vi "SaccadeAnalyser - Main.vi"(8 "error in (no error)":errorcluster, 11 "Data IN":T3={"Impulse Positions"=[{"Start"=5471, "End"=5813, "Impulse Plane"=enum."Yaw", "Impulse Direction +ve?"=FALSE, "Time offset"=0, "Amplitude offset"=0.0}, {"Start"=6974, "End"=7325, "Impulse Plane"=enum."Yaw", "Impulse Direction +ve?"=TRUE, "Time offset"=0, "Amplitude offset"=0.0}, {"Start"=7641, "End"=7980, "Impulse Plane"=enum."Yaw", "Impulse Direction +ve?"=FALSE, "Time offset"=0, "Amplitude offset"=0.0}, {"Start"=9060, "End"=9400, "Impulse Plane"=enum."Yaw", "Impulse Direction +ve?"=FALSE, "Time offset"=0, "Amplitude offset"=0.0}, {"Start"=9938, "End"=10282, "Impulse Plane"=enum."Yaw", "Impulse Direction +ve?"=FALSE, "Time offset"=0, "Amplitude offset"=0.0}, {"Start"=10800, "End"=11142, "Impulse Plane"=enum."Yaw", "Impulse Direction +ve?"=FALSE, "Time offset"=0, "Amplitude offset"=0.0}, {"Start"=11602, "End"=11942, "Impulse Plane"=enum."Yaw", "Impulse Direction +ve?"=TRUE, "Time offset"=0, "Amplitude offset"=0.0}, {"Start"=12449, "End"=12790, "Impulse Plane"=enum."Yaw", "Impulse Direction +ve?"=TRUE, "Time offset"=0, "Amplitude offset"=0.0}, {"Start"=13310, "End"=13653, "Impulse Plane"=enum."Yaw", "Impulse Direction +ve?"=TRUE, "Time offset"=0, "Amplitude offset"=0.0}, {"Start"=14191, "End"=14535, "Impulse Plane"=enum."Yaw", "Impulse Direction +ve?"=TRUE, "Time offset"=0, "Amplitude offset"=0.0}, {"Start"=15040, "End"=15380, "Impulse Plane"=enum."Yaw", "Impulse Direction +ve?"=FALSE, "Time offset"=0, "Amplitude offset"=0.0}, {"Start"=16780, "End"=17124, "Impulse Plane"=enum."Yaw", "Impulse Direction +ve?"=TRUE, "Time offset"=0, "Amplitude offset"=0.0}, {"Start"=17572, "End"=17913, "Impulse Plane"=enum."Yaw", "Impulse Direction +ve?"=FALSE, "Time offset"=0, "Amplitude offset"=0.0}, {"Start"=18369, "End"=18713, "Impulse Plane"=enum."Yaw", "Impulse Direction +ve?"=FALSE, "Time offset"=0, "Amplitude offset"=0.0}, {"Start"=19174, "End"=19519, "Impulse Plane"=enum."Yaw", "Impulse Direction +ve?"=FALSE, "Time offset"=0, "Amplitude offset"=0.0}, {"Start"=19928, "End"=20270, "Impulse Plane"=enum."Yaw", "Impulse Direction +ve?"=TRUE, "Time offset"=0, "Amplitude offset"=0.0}, {"Start"=20762, "End"=21121, "Impulse Plane"=enum."Yaw", "Impulse Direction +ve?"=FALSE, "Time offset"=0, "Amplitude offset"=0.0}, {"Start"=21554, "End"=21888, "Impulse Plane"=enum."Yaw", "Impulse Direction +ve?"=FALSE, "Time offset"=0, "Amplitude offset"=0.0}, {"Start"=22293, "End"=22639, "Impulse Plane"=enum."Yaw", "Impulse Direction +ve?"=TRUE, "Time offset"=0, "Amplitude offset"=0.0}, {"Start"=23109, "End"=23464, "Impulse Plane"=enum."Yaw", "Impulse Direction +ve?"=TRUE, "Time offset"=0, "Amplitude offset"=0.0}, {"Start"=23868, "End"=24215, "Impulse Plane"=enum."Yaw", "Impulse Direction +ve?"=TRUE, "Time offset"=0, "Amplitude offset"=0.0}, {"Start"=24643, "End"=24992, "Impulse Plane"=enum."Yaw", "Impulse Direction +ve?"=FALSE, "Time offset"=0, "Amplitude offset"=0.0}, {"Start"=25685, "End"=26023, "Impulse Plane"=enum."Yaw", "Impulse Direction +ve?"=FALSE, "Time offset"=0, "Amplitude offset"=0.0}, {"Start"=26431, "End"=26768, "Impulse Plane"=enum."Yaw", "Impulse Direction +ve?"=FALSE, "Time offset"=0, "Amplitude offset"=0.0}, {"Start"=27251, "End"=27595, "Impulse Plane"=enum."Yaw", "Impulse Direction +ve?"=FALSE, "Time offset"=0, "Amplitude offset"=0.0}, {"Start"=28832, "End"=29180, "Impulse Plane"=enum."Yaw", "Impulse Direction +ve?"=TRUE, "Time offset"=0, "Amplitude offset"=0.0}, {"Start"=31028, "End"=31383, "Impulse Plane"=enum."LARP", "Impulse Direction +ve?"=FALSE, "Time offset"=0, "Amplitude offset"=0.0}, {"Start"=32603, "End"=32936, "Impulse Plane"=enum."LARP", "Impulse Direction +ve?"=TRUE, "Time offset"=0, "Amplitude offset"=0.0}, {"Start"=33445, "End"=33779, "Impulse Plane"=enum."LARP", "Impulse Direction +ve?"=TRUE, "Time offset"=0, "Amplitude offset"=0.0}, {"Start"=34276, "End"=34629, "Impulse Plane"=enum."LARP", "Impulse Direction +ve?"=FALSE, "Time offset"=0, "Amplitude offset"=0.0}, {"Start"=35114, "End"=35460, "Impulse Plane"=enum."LARP", "Impulse Direction +ve?"=FALSE, "Time offset"=0, "Amplitude offset"=0.0}, {"Start"=35981, "End"=36324, "Impulse Plane"=enum."LARP", "Impulse Direction +ve?"=TRUE, "Time offset"=0, "Amplitude offset"=0.0}, {"Start"=36920, "End"=37249, "Impulse Plane"=enum."LARP", "Impulse Direction +ve?"=TRUE, "Time offset"=0, "Amplitude offset"=0.0}, {"Start"=37988, "End"=38322, "Impulse Plane"=enum."LARP", "Impulse Direction +ve?"=TRUE, "Time offset"=0, "Amplitude offset"=0.0}, {"Start"=38964, "End"=39324, "Impulse Plane"=enum."LARP", "Impulse Direction +ve?"=FALSE, "Time offset"=0, "Amplitude offset"=0.0}, {"Start"=39948, "End"=40284, "Impulse Plane"=enum."LARP", "Impulse Direction +ve?"=TRUE, "Time offset"=0, "Amplitude offset"=0.0}, {"Start"=40958, "End"=41293, "Impulse Plane"=enum."LARP", "Impulse Direction +ve?"=TRUE, "Time offset"=0, "Amplitude offset"=0.0}, {"Start"=41899, "End"=42229, "Impulse Plane"=enum."LARP", "Impulse Direction +ve?"=TRUE, "Time offset"=0, "Amplitude offset"=0.0}, {"Start"=42801, "End"=43154, "Impulse Plane"=enum."LARP", "Impulse Direction +ve?"=FALSE, "Time offset"=0, "Amplitude offset"=0.0}, {"Start"=43641, "End"=43980, "Impulse Plane"=enum."LARP", "Impulse Direction +ve?"=TRUE, "Time offset"=0, "Amplitude offset"=0.0}, {"Start"=44466, "End"=44821, "Impulse Plane"=enum."LARP", "Impulse Direction +ve?"=FALSE, "Time offset"=0, "Amplitude offset"=0.0}, {"Start"=45388, "End"=45722, "Impulse Plane"=enum."LARP", "Impulse Direction +ve?"=TRUE, "Time offset"=0, "Amplitude offset"=0.0}, {"Start"=46149, "End"=46510, "Impulse Plane"=enum."LARP", "Impulse Direction +ve?"=FALSE, "Time offset"=0, "Amplitude offset"=0.0}, {"Start"=47874, "End"=48206, "Impulse Plane"=enum."LARP", "Impulse Direction +ve?"=TRUE, "Time offset"=0, "Amplitude offset"=0.0}, {"Start"=50143, "End"=50479, "Impulse Plane"=enum."RALP", "Impulse Direction +ve?"=TRUE, "Time offset"=0, "Amplitude offset"=0.0}, {"Start"=50976, "End"=51310, "Impulse Plane"=enum."RALP", "Impulse Direction +ve?"=FALSE, "Time offset"=0, "Amplitude offset"=0.0}, {"Start"=51892, "End"=52226, "Impulse Plane"=enum."RALP", "Impulse Direction +ve?"=FALSE, "Time offset"=0, "Amplitude offset"=0.0}, {"Start"=52839, "End"=53171, "Impulse Plane"=enum."RALP", "Impulse Direction +ve?"=FALSE, "Time offset"=0, "Amplitude offset"=0.0}, {"Start"=53676, "End"=54012, "Impulse Plane"=enum."RALP", "Impulse Direction +ve?"=TRUE, "Time offset"=0, "Amplitude offset"=0.0}, {"Start"=54530, "End"=54877, "Impulse Plane"=enum."RALP", "Impulse Direction +ve?"=FALSE, "Time offset"=0, "Amplitude offset"=0.0}, {"Start"=55371, "End"=55711, "Impulse Plane"=enum."RALP", "Impulse Direction +ve?"=TRUE, "Time offset"=0, "Amplitude offset"=0.0}, {"Start"=56153, "End"=56482, "Impulse Plane"=enum."RALP", "Impulse Direction +ve?"=FALSE, "Time offset"=0, "Amplitude offset"=0.0}, {"Start"=57053, "End"=57390, "Impulse Plane"=enum."RALP", "Impulse Direction +ve?"=FALSE, "Time offset"=0, "Amplitude offset"=0.0}, {"Start"=57954, "End"=58292, "Impulse Plane"=enum."RALP", "Impulse Direction +ve?"=FALSE, "Time offset"=0, "Amplitude offset"=0.0}, {"Start"=58794, "End"=59130, "Impulse Plane"=enum."RALP", "Impulse Direction +ve?"=TRUE, "Time offset"=0, "Amplitude offset"=0.0}, {"Start"=59587, "End"=59931, "Impulse Plane"=enum."RALP", "Impulse Direction +ve?"=TRUE, "Time offset"=0, "Amplitude offset"=0.0}, {"Start"=60399, "End"=60744, "Impulse Plane"=enum."RALP", "Impulse Direction +ve?"=FALSE, "Time offset"=0, "Amplitude offset"=0.0}, {"Start"=61218, "End"=61559, "Impulse Plane"=enum."RALP", "Impulse Direction +ve?"=FALSE, "Time offset"=0, "Amplitude offset"=0.0}, {"Start"=62100, "End"=62442, "Impulse Plane"=enum."RALP", "Impulse Direction +ve?"=FALSE, "Time offset"=0, "Amplitude offset"=0.0}, {"Start"=62989, "End"=63322, "Impulse Plane"=enum."RALP", "Impulse Direction +ve?"=FALSE, "Time offset"=0, "Amplitude offset"=0.0}, {"Start"=63787, "End"=64136, "Impulse Plane"=enum."RALP", "Impulse Direction +ve?"=TRUE, "Time offset"=0, "Amplitude offset"=0.0}, {"Start"=64603, "End"=64953, "Impulse Plane"=enum."RALP", "Impulse Direction +ve?"=FALSE, "Time offset"=0, "Amplitude offset"=0.0}, {"Start"=65462, "End"=65795, "Impulse Plane"=enum."RALP", "Impulse Direction +ve?"=FALSE, "Time offset"=0, "Amplitude offset"=0.0}, {"Start"=66308, "End"=66645, "Impulse Plane"=enum."RALP", "Impulse Direction +ve?"=FALSE, "Time offset"=0, "Amplitude offset"=0.0}, {"Start"=67052, "End"=67402, "Impulse Plane"=enum."RALP", "Impulse Direction +ve?"=TRUE, "Time offset"=0, "Amplitude offset"=0.0}], "No. Imp"=15, "Parameter Time Series"=[{"time offset"=0.0, "Offset"=0.0, "Gain"=1.0, "inverse"=FALSE, "filter data"=FALSE, "dots"=FALSE, "interpolate"=FALSE, "List 1"=5, "Color Box"=6618880, "Boolean"=TRUE}, {"time offset"=0.0, "Offset"=0.0, "Gain"=1.0, "inverse"=FALSE, "filter data"=FALSE, "dots"=FALSE, "interpolate"=FALSE, "List 1"=6, "Color Box"=6618880, "Boolean"=FALSE}, {"time offset"=0.0, "Offset"=0.0, "Gain"=1.0, "inverse"=FALSE, "filter data"=FALSE, "dots"=FALSE, "interpolate"=FALSE, "List 1"=7, "Color Box"=6618880, "Boolean"=FALSE}, {"time offset"=0.0, "Offset"=0.0, "Gain"=1.0, "inverse"=FALSE, "filter data"=FALSE, "dots"=FALSE, "interpolate"=FALSE, "List 1"=13, "Color Box"=16777224, "Boolean"=TRUE}, {"time offset"=0.0, "Offset"=0.0, "Gain"=1.0, "inverse"=FALSE, "filter data"=FALSE, "dots"=FALSE, "interpolate"=FALSE, "List 1"=14, "Color Box"=16777224, "Boolean"=FALSE}, {"time offset"=0.0, "Offset"=0.0, "Gain"=1.0, "inverse"=FALSE, "filter data"=FALSE, "dots"=FALSE, "interpolate"=FALSE, "List 1"=15, "Color Box"=16777224, "Boolean"=FALSE}], "Parameter Impuls Series"=[{"Color"=6618880, "Visible"=TRUE, "Channel"=1, "Invert"=FALSE, "Desaccade"=FALSE, "Offset"=0.0, "Gain"=1.0}, {"Color"=6618880, "Visible"=FALSE, "Channel"=6, "Invert"=FALSE, "Desaccade"=FALSE, "Offset"=0.0, "Gain"=1.0}, {"Color"=6618880, "Visible"=FALSE, "Channel"=7, "Invert"=FALSE, "Desaccade"=FALSE, "Offset"=0.0, "Gain"=1.0}, {"Color"=16777224, "Visible"=TRUE, "Channel"=13, "Invert"=FALSE, "Desaccade"=FALSE, "Offset"=0.0, "Gain"=1.0}, {"Color"=16777224, "Visible"=FALSE, "Channel"=14, "Invert"=FALSE, "Desaccade"=FALSE, "Offset"=0.0, "Gain"=1.0}, {"Color"=16777224, "Visible"=FALSE, "Channel"=15, "Invert"=FALSE, "Desaccade"=FALSE, "Offset"=0.0, "Gain"=1.0}], "Experiment Parameters"={"Freq"=0.0, "Vel"=0, "Acc"=0, "Stimulus"="Head Impulse"}, "Autosort File"=refnum, "Data File"={"Data Channels"=array34x71049[2415666 elements], "Sample Rate"=500, "Channel List"=["Hz Position-in-Head", "Hz Velocity-in-Head", "Hy Position-in-Head", "Hy Velocity-in-Head", "Hx Position-in-Head", "Hx Velocity-in-Head", "Hl Velocity-in-Head", "Hr Velocity-in-Head", "Lx Position-in-Head", "Ly Position-in-Head", "Lz Position-in-Head", "Lx Velocity-in-Head", "Ly Velocity-in-Head", "Lz Velocity-in-Head", "Ll Velocity-in-Head", "Lr Velocity-in-Head", "Rx Position-in-Head", "Ry Position-in-Head", "Rz Position-in-Head", "Rx Velocity-in-Head", "Ry Velocity-in-Head", "Rz Velocity-in-Head", "Rl Velocity-in-Head", "Rr Velocity-in-Head", "Target on/off", "aux input 1", "aux input 2", " ", "", "", "", "Target Hor", "Target Ver", ""]}, "Experiment data path"=path "C:/Users/w.figtree/Desktop/Coils Data/3", "Image data path"=path "/Macintosh HD/Users/patrick/Studium/Diploma Thesis/Data Analysis", "LVS data path"=path "/Macintosh HD/Users/patrick/Studium/Diploma Thesis/Data Analysis", "Raw copy path"=path "/Macintosh HD/Users/patrick/Studium/Diploma Thesis/Data Analysis", "filename"="passive_lvs.lvs", "desaccading parameters"={"Tolerance"=3, "Acc Range"=7000.0, "Sample Rate"=500, "Impulse Plane 2"=enum."Yaw", "Impulse dir"=FALSE}, "Experiment Parameters 2"={"Subject"="SE Trial Short Term", "Strain"="", "Rotation plane"="", "Experimenter"=" ", "Trial"=0.0, "Time"=0.0}, "Excel"={"Excel._Application"=refnum, "Use Excel"=TRUE, "Worksheet SINE"=refnum, "Row SINE"=0, "Worksheet TRANS"=refnum, "Row TRANS"=0}, "Session Config File"=refnum, "Autosort Parameter Set"=4, "EMA Version"="EMA 2016a", "desacc "={"Threshold 1 [Acc]"=7000.0, "Threshold 2 [% of TH1]"=60, "tolerance"=3, "Search WD "=0.1, " always use TH2"=FALSE, "Range"=3.0, "Max time"=120.0, "Min time"=20.0, "Velocity Threshold"=150}, "Cycle Nr for Saccades"={"POS"=0, "NEG"=0}, "calibration name"="u_calibration_1_p00001s001_calib.mat", "Excel"=refnum} {"Parameter Time Series"."time offset" format="%.3f"; "Parameter Time Series"."Gain" format="%.1f"; "Parameter Time Series"."Offset" format="%.1f"; "Parameter Time Series"."List 1" items=["Motor-Pos", "Motor-Vel", "Lx Position-in-Head", "Ly Position-in-Head", "Lz Position-in-Head", "Lx Velocity-in-Head", "Ly Velocity-in-Head", "Lz Velocity-in-Head", "Ll Velocity-in-Head", "Lr Velocity-in-Head", "Lx Accel-in-Head", "Ly Accel-in-Head", "Lz Accel-in-Head", "Rx Position-in-Head", "Ry Position-in-Head", "Rz Position-in-Head", "Rx Velocity-in-Head", "Ry Velocity-in-Head", "Rz Velocity-in-Head", "Rl Velocity-in-Head", "Rr Velocity-in-Head", "Rx Accel-in-Head", "Ry Accel-in-Head", "Rz Accel-in-Head", "Global Trigger", "", "", ""]; "Parameter Impuls Series"."Gain" format="%.1f"; "Parameter Impuls Series"."Offset" format="%.1f"}) -> (0 "error out":errorcluster, 3 "Data OUT":T3={"Impulse Positions"=[{"Start"=5471, "End"=5813, "Impulse Plane"=enum."Yaw", "Impulse Direction +ve?"=FALSE, "Time offset"=0, "Amplitude offset"=0.0}, {"Start"=6974, "End"=7325, "Impulse Plane"=enum."Yaw", "Impulse Direction +ve?"=TRUE, "Time offset"=0, "Amplitude offset"=0.0}, {"Start"=7641, "End"=7980, "Impulse Plane"=enum."Yaw", "Impulse Direction +ve?"=FALSE, "Time offset"=0, "Amplitude offset"=0.0}, {"Start"=9060, "End"=9400, "Impulse Plane"=enum."Yaw", "Impulse Direction +ve?"=FALSE, "Time offset"=0, "Amplitude offset"=0.0}, {"Start"=9938, "End"=10282, "Impulse Plane"=enum."Yaw", "Impulse Direction +ve?"=FALSE, "Time offset"=0, "Amplitude offset"=0.0}, {"Start"=10800, "End"=11142, "Impulse Plane"=enum."Yaw", "Impulse Direction +ve?"=FALSE, "Time offset"=0, "Amplitude offset"=0.0}, {"Start"=11602, "End"=11942, "Impulse Plane"=enum."Yaw", "Impulse Direction +ve?"=TRUE, "Time offset"=0, "Amplitude offset"=0.0}, {"Start"=12449, "End"=12790, "Impulse Plane"=enum."Yaw", "Impulse Direction +ve?"=TRUE, "Time offset"=0, "Amplitude offset"=0.0}, {"Start"=13310, "End"=13653, "Impulse Plane"=enum."Yaw", "Impulse Direction +ve?"=TRUE, "Time offset"=0, "Amplitude offset"=0.0}, {"Start"=14191, "End"=14535, "Impulse Plane"=enum."Yaw", "Impulse Direction +ve?"=TRUE, "Time offset"=0, "Amplitude offset"=0.0}, {"Start"=15040, "End"=15380, "Impulse Plane"=enum."Yaw", "Impulse Direction +ve?"=FALSE, "Time offset"=0, "Amplitude offset"=0.0}, {"Start"=16780, "End"=17124, "Impulse Plane"=enum."Yaw", "Impulse Direction +ve?"=TRUE, "Time offset"=0, "Amplitude offset"=0.0}, {"Start"=17572, "End"=17913, "Impulse Plane"=enum."Yaw", "Impulse Direction +ve?"=FALSE, "Time offset"=0, "Amplitude offset"=0.0}, {"Start"=18369, "End"=18713, "Impulse Plane"=enum."Yaw", "Impulse Direction +ve?"=FALSE, "Time offset"=0, "Amplitude offset"=0.0}, {"Start"=19174, "End"=19519, "Impulse Plane"=enum."Yaw", "Impulse Direction +ve?"=FALSE, "Time offset"=0, "Amplitude offset"=0.0}, {"Start"=19928, "End"=20270, "Impulse Plane"=enum."Yaw", "Impulse Direction +ve?"=TRUE, "Time offset"=0, "Amplitude offset"=0.0}, {"Start"=20762, "End"=21121, "Impulse Plane"=enum."Yaw", "Impulse Direction +ve?"=FALSE, "Time offset"=0, "Amplitude offset"=0.0}, {"Start"=21554, "End"=21888, "Impulse Plane"=enum."Yaw", "Impulse Direction +ve?"=FALSE, "Time offset"=0, "Amplitude offset"=0.0}, {"Start"=22293, "End"=22639, "Impulse Plane"=enum."Yaw", "Impulse Direction +ve?"=TRUE, "Time offset"=0, "Amplitude offset"=0.0}, {"Start"=23109, "End"=23464, "Impulse Plane"=enum."Yaw", "Impulse Direction +ve?"=TRUE, "Time offset"=0, "Amplitude offset"=0.0}, {"Start"=23868, "End"=24215, "Impulse Plane"=enum."Yaw", "Impulse Direction +ve?"=TRUE, "Time offset"=0, "Amplitude offset"=0.0}, {"Start"=24643, "End"=24992, "Impulse Plane"=enum."Yaw", "Impulse Direction +ve?"=FALSE, "Time offset"=0, "Amplitude offset"=0.0}, {"Start"=25685, "End"=26023, "Impulse Plane"=enum."Yaw", "Impulse Direction +ve?"=FALSE, "Time offset"=0, "Amplitude offset"=0.0}, {"Start"=26431, "End"=26768, "Impulse Plane"=enum."Yaw", "Impulse Direction +ve?"=FALSE, "Time offset"=0, "Amplitude offset"=0.0}, {"Start"=27251, "End"=27595, "Impulse Plane"=enum."Yaw", "Impulse Direction +ve?"=FALSE, "Time offset"=0, "Amplitude offset"=0.0}, {"Start"=28832, "End"=29180, "Impulse Plane"=enum."Yaw", "Impulse Direction +ve?"=TRUE, "Time offset"=0, "Amplitude offset"=0.0}, {"Start"=31028, "End"=31383, "Impulse Plane"=enum."LARP", "Impulse Direction +ve?"=FALSE, "Time offset"=0, "Amplitude offset"=0.0}, {"Start"=32603, "End"=32936, "Impulse Plane"=enum."LARP", "Impulse Direction +ve?"=TRUE, "Time offset"=0, "Amplitude offset"=0.0}, {"Start"=33445, "End"=33779, "Impulse Plane"=enum."LARP", "Impulse Direction +ve?"=TRUE, "Time offset"=0, "Amplitude offset"=0.0}, {"Start"=34276, "End"=34629, "Impulse Plane"=enum."LARP", "Impulse Direction +ve?"=FALSE, "Time offset"=0, "Amplitude offset"=0.0}, {"Start"=35114, "End"=35460, "Impulse Plane"=enum."LARP", "Impulse Direction +ve?"=FALSE, "Time offset"=0, "Amplitude offset"=0.0}, {"Start"=35981, "End"=36324, "Impulse Plane"=enum."LARP", "Impulse Direction +ve?"=TRUE, "Time offset"=0, "Amplitude offset"=0.0}, {"Start"=36920, "End"=37249, "Impulse Plane"=enum."LARP", "Impulse Direction +ve?"=TRUE, "Time offset"=0, "Amplitude offset"=0.0}, {"Start"=37988, "End"=38322, "Impulse Plane"=enum."LARP", "Impulse Direction +ve?"=TRUE, "Time offset"=0, "Amplitude offset"=0.0}, {"Start"=38964, "End"=39324, "Impulse Plane"=enum."LARP", "Impulse Direction +ve?"=FALSE, "Time offset"=0, "Amplitude offset"=0.0}, {"Start"=39948, "End"=40284, "Impulse Plane"=enum."LARP", "Impulse Direction +ve?"=TRUE, "Time offset"=0, "Amplitude offset"=0.0}, {"Start"=40958, "End"=41293, "Impulse Plane"=enum."LARP", "Impulse Direction +ve?"=TRUE, "Time offset"=0, "Amplitude offset"=0.0}, {"Start"=41899, "End"=42229, "Impulse Plane"=enum."LARP", "Impulse Direction +ve?"=TRUE, "Time offset"=0, "Amplitude offset"=0.0}, {"Start"=42801, "End"=43154, "Impulse Plane"=enum."LARP", "Impulse Direction +ve?"=FALSE, "Time offset"=0, "Amplitude offset"=0.0}, {"Start"=43641, "End"=43980, "Impulse Plane"=enum."LARP", "Impulse Direction +ve?"=TRUE, "Time offset"=0, "Amplitude offset"=0.0}, {"Start"=44466, "End"=44821, "Impulse Plane"=enum."LARP", "Impulse Direction +ve?"=FALSE, "Time offset"=0, "Amplitude offset"=0.0}, {"Start"=45388, "End"=45722, "Impulse Plane"=enum."LARP", "Impulse Direction +ve?"=TRUE, "Time offset"=0, "Amplitude offset"=0.0}, {"Start"=46149, "End"=46510, "Impulse Plane"=enum."LARP", "Impulse Direction +ve?"=FALSE, "Time offset"=0, "Amplitude offset"=0.0}, {"Start"=47874, "End"=48206, "Impulse Plane"=enum."LARP", "Impulse Direction +ve?"=TRUE, "Time offset"=0, "Amplitude offset"=0.0}, {"Start"=50143, "End"=50479, "Impulse Plane"=enum."RALP", "Impulse Direction +ve?"=TRUE, "Time offset"=0, "Amplitude offset"=0.0}, {"Start"=50976, "End"=51310, "Impulse Plane"=enum."RALP", "Impulse Direction +ve?"=FALSE, "Time offset"=0, "Amplitude offset"=0.0}, {"Start"=51892, "End"=52226, "Impulse Plane"=enum."RALP", "Impulse Direction +ve?"=FALSE, "Time offset"=0, "Amplitude offset"=0.0}, {"Start"=52839, "End"=53171, "Impulse Plane"=enum."RALP", "Impulse Direction +ve?"=FALSE, "Time offset"=0, "Amplitude offset"=0.0}, {"Start"=53676, "End"=54012, "Impulse Plane"=enum."RALP", "Impulse Direction +ve?"=TRUE, "Time offset"=0, "Amplitude offset"=0.0}, {"Start"=54530, "End"=54877, "Impulse Plane"=enum."RALP", "Impulse Direction +ve?"=FALSE, "Time offset"=0, "Amplitude offset"=0.0}, {"Start"=55371, "End"=55711, "Impulse Plane"=enum."RALP", "Impulse Direction +ve?"=TRUE, "Time offset"=0, "Amplitude offset"=0.0}, {"Start" (continued)
    shift-left: T6 {"Impulse Data"=refnum, "Sample Rate (Hz)"=0.0, "Num Impulses"=0, "Impulse Duration (samples)"=0, "Palette"={"Stimulus"=6618880, "Response"=16777224, "Saccade"=16777224, "Excluded Saccade"=16777224, "Sibling Saccade"=16777224, "Selected Saccade"=16777224}, "Saccades"=[], "Summary"={"Num Impulses"=0.0, "Num Saccades"=0.0, "Onset (ms)"=0.0, "Onset SD (ms)"=0.0, "Duration (ms)"=0.0, "Duration SD (ms)"=0.0, "Vel (°/s)"=0.0, "Vel SD (°/s)"=0.0, "Amplitude (°)"=0.0, "Amplitude SD (°)"=0.0, "Gain"=0.0, "Gain SD"=0.0}, "Group Summary"=[]} ("Saccade Analyser Data") -> [w121]
    stop <- w126 stop-if-true
    # "Main Loop"
    n86 = Dequeue Element(queue=w129) -> (queue out=w128:refnum<queue>, element=w127:T10)  [unwired: 2 in, 2 out]
    n87 = case shown="\"Export - Saccades\"" w127 {
      tunnel: w128 -> [_ w158 _ w180 w187 _ _ _ _ _ _ w464 _ _ _ _ _ _ _ _ _ _ _ _ _ w702 w709 w715 _ _ _ _ _ _ w900]
      tunnel: [_ _ TRUE _ _ _ _ _ _ _ _ _ _ _ _ _ _ _ _ _ _ _ _ _ _ _ _ _ _ _ _ _ _ _ _] -> w126
      tunnel: w125 -> [w132 w156 w177 w183 w190 w219 w236 w279 w328 w369 w409 w467 w473 w487 w521 w572 w598 w622 w661 w667 w673 w678 w685 w689 w696 w705 w712 w719 w724 w745 w773 w789 w829 w839 w904]
      tunnel: w124 -> [w131 w162 w176 w182 w189 w220 w235 w278 w327 w368 w408 w466 w472 w486 w520 w571 w597 w621 w660 w666 w672 w677 w684 w688 w695 w704 w711 w718 w733 w770 w782 w810 w837 w864 w903]
      tunnel: [w132 w156 w177 w183 w190 w219 w236 w279 w328 w369 w409 w467 w473 w487 w521 w572 w598 w622 w661 w667 w673 w678 w685 w689 w696 w705 w712 w719 w723 w744 w772 w790 w830 w841 w904] -> w123
      tunnel: [w131 w162 w176 w182 w189 w220 w235 w278 w327 w368 w408 w466 w472 w486 w520 w571 w597 w621 w660 w666 w672 w677 w684 w688 w695 w704 w711 w718 w733 w770 w782 w810 w837 w864 w903] -> w122
      tunnel: w121 -> [w130 w161 w175 w181 w188 w215 w234 w276 w326 w367 w405 w465 w471 w481 w508 w570 w596 w620 w658 w665 w671 w676 w683 w687 w692 w703 w710 w717 w722 w735 w771 w791 w828 w840 w902]
      tunnel: [w130 w160 w175 w181 w188 w213 w234 w275 w325 w366 w404 w465 w471 w481 w508 w570 w596 w620 w658 w665 w671 w676 w683 w687 w691 w703 w710 w717 w722 w735 w771 w791 w828 w840 w902] -> w120
      frame Default {
        # "Unhandled state. Should never occur."
        n88 = One Button Dialog(message="Error: Unhandled state in Saccade Analyser!") -> ()  [unwired: 1 in, 1 out]
      }
      frame "Initialise" {
        w137 = u16 10 items=["Hz Position-in-Head", "Hz Velocity-in-Head", "Hy Position-in-Head", "Hy Velocity-in-Head", "Hx Position-in-Head", "Hx Velocity-in-Head", "Hl Velocity-in-Head", "Hr Velocity-in-Head", "Lx Position-in-Head", "Ly Position-in-Head", "Lz Position-in-Head", "Lx Velocity-in-Head", "Ly Velocity-in-Head", "Lz Velocity-in-Head", "Ll Velocity-in-Head", "Lr Velocity-in-Head", "Rx Position-in-Head", "Ry Position-in-Head", "Rz Position-in-Head", "Rx Velocity-in-Head", "Ry Velocity-in-Head", "Rz Velocity-in-Head", "Rl Velocity-in-Head", "Rr Velocity-in-Head", "Target on/off", "aux input 1", "aux input 2", " ", "", "", "", "Target Hor", "Target Ver", ""] ("ring_response channel")
        w146 = u16 13 items=["Hz Position-in-Head", "Hz Velocity-in-Head", "Hy Position-in-Head", "Hy Velocity-in-Head", "Hx Position-in-Head", "Hx Velocity-in-Head", "Hl Velocity-in-Head", "Hr Velocity-in-Head", "Lx Position-in-Head", "Ly Position-in-Head", "Lz Position-in-Head", "Lx Velocity-in-Head", "Ly Velocity-in-Head", "Lz Velocity-in-Head", "Ll Velocity-in-Head", "Lr Velocity-in-Head", "Rx Position-in-Head", "Ry Position-in-Head", "Rz Position-in-Head", "Rx Velocity-in-Head", "Ry Velocity-in-Head", "Rz Velocity-in-Head", "Rl Velocity-in-Head", "Rr Velocity-in-Head", "Target on/off", "aux input 1", "aux input 2", " ", "", "", "", "Target Hor", "Target Ver", ""] ("ring_response channel")
        w145 = u16 1 items=["Hz Position-in-Head", "Hz Velocity-in-Head", "Hy Position-in-Head", "Hy Velocity-in-Head", "Hx Position-in-Head", "Hx Velocity-in-Head", "Hl Velocity-in-Head", "Hr Velocity-in-Head", "Lx Position-in-Head", "Ly Position-in-Head", "Lz Position-in-Head", "Lx Velocity-in-Head", "Ly Velocity-in-Head", "Lz Velocity-in-Head", "Ll Velocity-in-Head", "Lr Velocity-in-Head", "Rx Position-in-Head", "Ry Position-in-Head", "Rz Position-in-Head", "Rx Velocity-in-Head", "Ry Velocity-in-Head", "Rz Velocity-in-Head", "Rl Velocity-in-Head", "Rr Velocity-in-Head", "Target on/off", "aux input 1", "aux input 2", " ", "", "", "", "Target Hor", "Target Ver", ""] ("ring_stimulus channel")
        # "LARP and RALP position are unfortunately not included in EMAs default data set. Since this plugin needs this data it will calculate it from the xyz data. In order to present a unified interface the channels are included in the UI list here."
        # "Configure VI for execution."
        n89 = control-ref of="mclb_saccades"() -> (w138:refnum<vi>)
        n90 = Enqueue Element(queue=w158, element=Saccade_Analyser_States."DO - Analysis") -> ()  [unwired: 2 in, 3 out]
        n91 = local write "Tab Control"(enum32{"Channel Select", "Detection", "Gain"}."Channel Select" ("Tab Control")) -> ()
        n92 = local write "enum_direction"(enum16{"Positive", "Negative"}."Positive" ("enum_direction")) -> ()
        n93 = local write "enum_plane"(T14."Yaw" ("enum_plane")) -> ()
        n94 = property on="Property Node" class="MCListbox (strict)"(reference=w138, "Key Focus"=TRUE) -> ()  [unwired: 1 in, 2 out]
        n95 = local write "ring_stimulusChannel"(w145) -> ()
        n96 = local write "ring_responseChannel"(w146) -> ()
        n97 = local write "ring_responsePosChannel"(w137) -> ()
        n98 = disable-structure shown="Disabled" {
          frame Disabled {
            # "Initialise analysis configuration. Disabled to allow value persistence between dialog calls."
            n99 = local write "sac_NSampleTime"(u32 10 ("sac_NSamples")) -> ()
            n100 = local write "bool_includePrePeak"(TRUE ("bool_includePrePeak")) -> ()
            n101 = local write "stim_Onset%"(4.0 ("Impulse Onset %")) -> ()
            n102 = local write "sac_BiphasicCond"(1.5 ("sac_BiphasicCond")) -> ()
            n103 = local write "sac_AccMult"(1.3 ("sac_AccMult")) -> ()
            n104 = local write "sac_AccMin"(2000.0 ("sac_AccMin")) -> ()
            n105 = local write "bool_autoChannel"(TRUE ("bool_autoChannel")) -> ()
            n106 = local write "enum_summaryType"(enum16{"Mean", "Median"}."Mean" ("enum_summaryType")) -> ()
            n107 = local write "gain_WinDur"(30.0 ("gain_WinDur")) -> ()
            n108 = local write "gain_WinLead"(40.0 ("gain_WinLead")) -> ()
            n109 = local write "gain_Valid%"(50.0 ("gain_ Valid%")) -> ()
          }
          frame Enabled {
          }
        }
        n110 = Unbundle By Name(w156) -> ("Data File.Sample Rate"=w159:i32, "Data File.Channel List"=w136:string[])
        n111 = Build Array (concatenate)(w136, string[] ["Ll Position-in-Head", "Lr Position-in-Head"] ("element")) -> (w135:string[])
        n112 = property on="ring_stimulusChannel" class="Ring (strict)"("Strings []"=w135) -> ()  [unwired: 2 in, 2 out]
        n113 = property on="ring_responsePosChannel" class="Ring (strict)"("Strings []"=w135) -> ()  [unwired: 2 in, 2 out]
        n114 = property on="ring_responseChannel" class="Ring (strict)"("Strings []"=w135) -> ()  [unwired: 2 in, 2 out]
        n115 = Bundle By Name(cluster=T7 {"Stimulus"=6618880, "Response"=16777224, "Saccade"=16777224, "Excluded Saccade"=16777224, "Sibling Saccade"=16777224, "Selected Saccade"=16777224} ("Palette"), "Stimulus"=u32 122893, "Response"=u32 16777224, "Saccade"=u32 16728128, "Excluded Saccade"=u32 9868950, "Sibling Saccade"=u32 16728128, "Selected Saccade"=u32 16728128) -> (w143:T7)
        n116 = New Data Value Reference(data value=T15[] []) -> (data value reference=w151:refnum<data-value>)  [unwired: 1 in, 1 out]
        n117 = Bundle By Name(cluster=w161, "Impulse Data"=w151, "Sample Rate (Hz)"=w159, "Palette"=w143, "Saccades"=T8[] []) -> (w160:T6)
      }
      frame "Quit" {
        # "End VI execution."
        n118 = Unbundle By Name(w175) -> ("Impulse Data"=w174:refnum<data-value>)
        n119 = Delete Data Value Reference(data value reference=w174) -> ()  [unwired: 1 in, 2 out]
      }
      frame "DO - Analysis" {
        w179 = T10[] [enum."Halt Panel Updates", enum."Disable Controls", enum."Load Channel Data", enum."Find Impulses", enum."Find Saccades", enum."Sequence Saccades", enum."Calc Saccade Summary Stats", enum."Calc Saccade Group Stats", enum."DO - Draw"] items=["Initialise", "Quit", "DO - Analysis", "DO - Summary Analysis", "Load Channel Data", "Find Impulses", "Find Saccades", "Sequence Saccades", "Calc Saccade Summary Stats", "Calc Saccade Group Stats", "DO - Draw", "Clear Plot", "Plot Selected Saccade", "Plot Selected Saccade Siblings", "Plot Impulse Data", "Plot Saccade Data", "Fill Saccade MCLB", "Fill Summary Stats", "Give MCLB Focus", "Halt Panel Updates", "Resume Panel Updates", "Disable Controls", "Enable Controls", "Toggle Saccade", "DO - Export Summary", "Export - Open Summary", "Export - Summary", "DO - Export Saccades", "Export - Open Saccades", "Export - Saccades", "DO - Export Group", "Export - Open Group", "Export - Group", "Do - Export All"] ("element")
        # "Enqueue analysis process states."
        n120 = for {
          tunnel: w180 -> [w185]
          tunnel: w179 -> [w184] mode=indexing
          n121 = Enqueue Element(queue=w185, element=w184) -> ()  [unwired: 2 in, 3 out]
        }
      }
      frame "DO - Summary Analysis" {
        w186 = T10[] [enum."Halt Panel Updates", enum."Disable Controls", enum."Sequence Saccades", enum."Calc Saccade Summary Stats", enum."Calc Saccade Group Stats", enum."DO - Draw"] items=["Initialise", "Quit", "DO - Analysis", "DO - Summary Analysis", "Load Channel Data", "Find Impulses", "Find Saccades", "Sequence Saccades", "Calc Saccade Summary Stats", "Calc Saccade Group Stats", "DO - Draw", "Clear Plot", "Plot Selected Saccade", "Plot Selected Saccade Siblings", "Plot Impulse Data", "Plot Saccade Data", "Fill Saccade MCLB", "Fill Summary Stats", "Give MCLB Focus", "Halt Panel Updates", "Resume Panel Updates", "Disable Controls", "Enable Controls", "Toggle Saccade", "DO - Export Summary", "Export - Open Summary", "Export - Summary", "DO - Export Saccades", "Export - Open Saccades", "Export - Saccades", "DO - Export Group", "Export - Open Group", "Export - Group", "Do - Export All"] ("element")
        # "Enqueue only the summary analysis process states."
        n122 = for {
          tunnel: w187 -> [w192]
          tunnel: w186 -> [w191] mode=indexing
          n123 = Enqueue Element(queue=w192, element=w191) -> ()  [unwired: 2 in, 3 out]
        }
      }
      frame "Load Channel Data" {
        # "Build Impulse Filter"
        # "Get Impulse Data"
        # "Load channel data from Data IN and sort them into impulses."
        n124 = property on="ring_responsePosChannel" class="Ring (strict)"() -> ("Strings []"=w195:string[], "Value"=w196:u16)  [unwired: 2 in, 2 out]
        n125 = property on="ring_stimulusChannel" class="Ring (strict)"() -> ("Strings []"=w207:string[], "Value"=w206:u16)  [unwired: 2 in, 2 out]
        n126 = property on="ring_responseChannel" class="Ring (strict)"() -> ("Strings []"=w205:string[], "Value"=w204:u16)  [unwired: 2 in, 2 out]
        n127 = local read "enum_direction"() -> (w211:enum16{"Positive", "Negative"})
        n128 = local read "enum_plane"() -> (w208:T2)
        n129 = Index Array(array=w207, index=w206) -> (element=w203:string)
        n130 = Index Array(array=w195, index=w196) -> (element=w194:string)
        n131 = Index Array(array=w205, index=w204) -> (element=w202:string)
        n132 = Build Array(w203, w202, w194) -> (w201:string[])
        n133 = Equal To 0?(x=w211) -> (x = 0?=w210:bool)
        n134 = Bundle By Name(cluster=T16 {"Channels"=["Hz Velocity-in-Head", "Lz Velocity-in-Head"], "Impulse Plane"=enum."Yaw", "Impulse Direction +ve?"=TRUE} ("Impulse Select"), "Channels"=w201, "Impulse Plane"=w208, "Impulse Direction +ve?"=w210) -> (w209:T16)
        n135 = Unbundle By Name(w219) -> ("Data File"=w218:T19, "Impulse Positions"=w217:T20)
        n136 = local read "bool_isCoilsData"() -> (w193:bool)
        n137 = call "Sort Impulses.vi"("Is Coils Data?"=w193, "Impulse Select"=w209, "Impulse Positions"=w217, "Data Input"=w218) -> ("Num Impulses"=w198:i32, "Impulses Duration (samples)"=w197:i32, "Impulse Data"=w200:dbl[][])  [unwired: 4 in, 1 out]
        n138 = for {
          N: w198 -> [_]
          tunnel: w200 -> [w229]
          tunnel: w198 -> [w221]
          tunnel: [w227] -> w199 mode=indexing
          i -> [w223]
          # "Collect data into impulse clusters\nData is organised by row first by impulse index then by channel index."
          n139 = Add(x=w223, y=w221) -> (x+y=w222:i32)
          n140 = Add(x=w222, y=w221) -> (x+y=w224:i32)
          n141 = Index Array(array=w229, index (row) #1=w223, index (row) #2=w222, index (row) #3=w224) -> (element #1=w228:dbl[], element #2=w226:dbl[], element #3=w225:dbl[])  [unwired: 3 in]
          n142 = Bundle By Name(cluster=T15 {"Stimulus Data"=[], "Response Data"=[], "Response Pos Data"=[], "Peak (idx)"=0, "Onset (idx)"=0} ("Impulse"), "Stimulus Data"=w228, "Response Data"=w226, "Response Pos Data"=w225) -> (w227:T15)
        }
        n143 = Unbundle By Name(w215) -> ("Impulse Data"=w216:refnum<data-value>)
        n144 = in-place {
          in-place-border: w199 -> [w231]
          n145 = in-place-dvr #1(w216) -> ()  [unwired: 2 out]
          n146 = in-place-dvr #1(w231) -> (w214:refnum<data-value>)  [unwired: 1 out]
        }
        n147 = Bundle By Name(cluster=w215, "Num Impulses"=w198, "Impulse Duration (samples)"=w197, "Impulse Data"=w214) -> (w213:T6)
      }
      frame "Find Impulses" {
        # "Finds the onset and peak of each impulse."
        n148 = Unbundle By Name(w234) -> ("Impulse Data"=w233:refnum<data-value>)
        n149 = local read "enum_direction"() -> (w232:enum16{"Positive", "Negative"})
        n150 = in-place {
          in-place-border: w232 -> [w237]
          n151 = in-place-dvr #2(w233) -> (w239:T15[])  [unwired: 1 out]
          n152 = for {
            tunnel: w239 -> [w246] mode=indexing
            tunnel: [w245] -> w238 mode=indexing
            tunnel: w237 -> [w241]
            # "Smooth signal"
            # "Find onset"
            # "Find Peak"
            # "For each impulse..."
            n153 = Unbundle By Name(w246) -> ("Stimulus Data"=w242:dbl[])
            n154 = call "SaccadeAnalyser - Make Traces Positive.vi"("enum_direction"=w241, "Stimulus in"=w242) -> ("Stimulus out"=w240:dbl[])  [unwired: 7 in, 2 out]
            n155 = Array Max & Min(array=w240) -> (max value=w253:dbl, max index (indices)=w244:i32)  [unwired: 2 out]
            n156 = local read "stim_Onset%"() -> (w255:dbl)
            n157 = call <vilib>:"Median Filter.vi"("left rank"=10, "X"=w240) -> ("Filtered X"=w248:dbl[])  [unwired: 8 in, 1 out]
            n158 = Divide(x=w255, y=100.0) -> (x/y=w252:dbl)
            n159 = Multiply(x=w253, y=w252) -> (x*y=w251:dbl)
            n160 = Greater?(x=w248, y=w251) -> (0:w250:bool[])
            n161 = Search 1D Array(1D array=w250, element=TRUE) -> (index of element=w243:i32)  [unwired: 1 in]
            n162 = Bundle By Name(cluster=w246, "Peak (idx)"=w244, "Onset (idx)"=w243) -> (w245:T15)
          }
          n163 = in-place-dvr #2(w238) -> ()  [unwired: 2 out]
        }
      }
      frame "Find Saccades" {
        # "Finds the saccades within each impulse and calculates the saccade onset, peak, duration, etc..."
        n164 = local read "enum_direction"() -> (w269:enum16{"Positive", "Negative"})
        n165 = Unbundle By Name(w276) -> ("Impulse Data"=w277:refnum<data-value>, "Sample Rate (Hz)"=w265:dbl)
        n166 = in-place {
          in-place-border: w265 -> [w283]
          in-place-border: [w282] -> w274
          in-place-border: w269 -> [w281]
          n167 = in-place-dvr #3(w277) -> (w285:T15[])  [unwired: 1 out]
          n168 = for {
            tunnel: w285 -> [w303] mode=indexing
            tunnel: [w303] -> w284 mode=indexing
            tunnel: w283 -> [w289]
            tunnel: [w301] -> w282 mode=concatenating
            tunnel: w281 -> [w300]
            i -> [w302]
            # "For each impulse..."
            n169 = Unbundle By Name(w303) -> ("Peak (idx)"=w286:i32, "Onset (idx)"=w298:i32, "Response Data"=w299:dbl[])
            n170 = local read "sac_NSampleTime"() -> (w294:dbl)
            n171 = local read "sac_BiphasicCond"() -> (w295:dbl)
            n172 = local read "bool_includePrePeak"() -> (w287:bool)
            n173 = local read "sac_AccMult"() -> (w296:dbl)
            n174 = local read "sac_AccMin"() -> (w297:dbl)
            n175 = Divide(x=w294, y=1000.0) -> (x/y=w293:dbl)
            n176 = call "SaccadeAnalyser - Make Traces Positive.vi"("enum_direction"=w300, "Response in"=w299) -> ("Response out"=w290:dbl[])  [unwired: 7 in, 2 out]
            n177 = Bundle(w293, "sac_AccMin"=w297, "sac_AccMult"=w296, "sac_BiphasicCond"=w295) -> (w288:T21)  [unwired: 1 in]
            n178 = call "Detect Saccades 2.vi"("Config"=w288, "Sample Rate (Hz)"=w289, "Velocity Data"=w290) -> ("Saccades"=w291:T8[])  [unwired: 7 in, 1 out]
            n179 = for {
              tunnel: [w315] -> w301 mode=indexing if=w309
              tunnel: w302 -> [w311]
              tunnel: w291 -> [w313] mode=indexing
              tunnel: w298 -> [w312]
              tunnel: w287 -> [w305]
              tunnel: w286 -> [w307]
              # "Check saccade is post onset"
              # "Check saccade is post peak"
              # "Remove early saccades and fill in basic info"
              n180 = Unbundle By Name(w313) -> ("Start (idx)"=w308:dbl)
              n181 = Bundle By Name(cluster=w313, "Impulse"=w311, "Included?"=TRUE) -> (w315:T8)
              n182 = Greater?(x=w308, y=w312) -> (0:w310:bool)
              n183 = Greater?(x=w308, y=w307) -> (0:w306:bool)
              n184 = Compound Arithmetic op=OR(w305, w306) -> (w304:bool)
              n185 = Compound Arithmetic op=AND(w304, w310) -> (w309:bool)
            }
          }
          n186 = in-place-dvr #3(w284) -> (w266:refnum<data-value>, w280:errorcluster)
        }
        n187 = call "Detect Saccade Peak.vi"("enum_direction"=w269, "Impulse Data"=w266, "error in (no error)"=w280, "Saccades in"=w274) -> ("error out"=w272:errorcluster, "Saccade out"=w273:T8[])  [unwired: 4 in]
        n188 = call "Trim Saccade Tail for Symmetry.vi"("error in (no error)"=w272, "Saccades in"=w273) -> ("error out"=w270:errorcluster, "Saccades out"=w271:T8[])  [unwired: 8 in]
        n189 = local read "gain_WinLead"() -> (w260:dbl)
        n190 = local read "gain_WinDur"() -> (w259:dbl)
        n191 = local read "gain_Valid%"() -> (w263:dbl)
        n192 = Bundle("gain_WinLead"=w260, "gain_WinDur"=w259) -> (w258:cluster{"gain_WinLead":dbl, "gain_WinDur":dbl})  [unwired: 1 in]
        n193 = call "Calculate Saccade Parameters.vi"("Impulse Data"=w266, "error in (no error)"=w270, "Sample Rate (Hz)"=w265, "enum_direction"=w269, "Saccades in"=w271) -> ("error out"=w267:errorcluster, "Saccade out"=w268:T8[])  [unwired: 5 in]
        n194 = Divide(x=w263, y=100.0) -> (x/y=w261:dbl)
        n195 = Divide(x=w258, y=1000.0) -> (x/y=w256:cluster{"gain_WinLead":dbl, "gain_WinDur":dbl})
        n196 = call "Calculate Saccade Gain.vi"("Gain Window"=w256, "Impulse Data"=w266, "error in (no error)"=w267, "Sample Rate (Hz)"=w265, "Valid Range Fraction"=w261, "Saccades in"=w268) -> ("Saccade out"=w264:T8[])  [unwired: 4 in, 1 out]
        n197 = Bundle By Name(cluster=w276, "Saccades"=w264) -> (w275:T6)
      }
      frame "Sequence Saccades" {
        w323 = u16 0 items=["Real, Imaginary", "Magnitude, Real, Imaginary", "Magnitude, Phase Angle"] ("method")
        # "Sort array. First by Impulse number (real) and then by onset index (imaginary)."
        # "Determines the order in which saccades appear within an impulse."
        n198 = Unbundle By Name(w326) -> ("Saccades"=w322:T8[])
        n199 = for {
          tunnel: w322 -> [w345] mode=indexing
          tunnel: [w343] -> w321 mode=indexing
          # "Initialise sequence number to NaN."
          n200 = Bundle By Name(cluster=w345, "Sequence #"=nan) -> (w343:T8)
        }
        n201 = for {
          tunnel: w321 -> [w351] mode=indexing
          tunnel: [w348] -> w324 mode=indexing if=w346
          tunnel: [w347] -> w320 mode=indexing if=w346
          i -> [w347]
          # "Get included saccades and build sorting array."
          n202 = Unbundle By Name(w351) -> ("Impulse"=w350:i32, "Start (idx)"=w349:dbl, "Included?"=w346:bool)
          n203 = Re/Im To Complex(1:w349, 2:w350) -> (0:w348:cdb)
        }
        n204 = call <vilib>:"Sort Complex Numbers.vi"("method"=w323, "Complex Numbers"=w324) -> ("Sorted Index"=w319:i32[])  [unwired: 7 in, 2 out]
        n205 = call-poly <userlib>:"Reorder Array2__ogtk.vi"("indices"=w319, "array"=w320) -> ("reordered array"=w318:i32[])  [unwired: 9 in]
        n206 = for {
          tunnel: w318 -> [w332] mode=indexing
          shift-right: [w331] -> w317
          shift-left: w321 -> [w333]
          shift-right: [FALSE] -> _
          shift-left: TRUE -> [w330]
          # "For each ordered and included saccade determine the sequence number"
          n207 = in-place {
            in-place-border: w330 -> [w334]
            n208 = in-place-array #4(w333, w332) -> (w340:T8)
            n209 = Unbundle By Name(w340) -> ("Impulse"=w342:i32)
            n210 = call-poly <userlib>:"Data Changed__ogtk.vi"("I32"=w342) -> ("Changed"=w336:bool)
            n211 = Compound Arithmetic op=OR(w336, w334) -> (w335:bool)
            n212 = call <vilib>:"Increment PtByPt.vi"("initialize"=w335, "activate"=TRUE) -> ("counter"=w339:u32)  [unwired: 1 out]
            n213 = Decrement(x=w339) -> (x-1=w337:u32)
            n214 = Bundle By Name(cluster=w340, "Sequence #"=w337) -> (w338:T8)
            n215 = in-place-array #4(w338) -> (w331:T8[])  [unwired: 1 out]
          }
        }
        n216 = Bundle By Name(cluster=w326, "Saccades"=w317) -> (w325:T6)
      }
      frame "Calc Saccade Summary Stats" {
        # "Calculates the summary statistics across all the saccades."
        n217 = Unbundle By Name(w367) -> ("Saccades"=w365:T8[])
        n218 = for {
          tunnel: w365 -> [w402] mode=indexing
          tunnel: [w396] -> w363 mode=indexing if=w394
          tunnel: [w395] -> w360 mode=indexing if=w394
          # "Gather stats to be summarised from each saccade."
          n219 = Unbundle By Name(w402) -> ("Onset (ms)"=w401:dbl, "Duration (ms)"=w400:dbl, "Vel (°/s)"=w399:dbl, "Amplitude (°)"=w398:dbl, "Gain"=w397:dbl, "Included?"=w394:bool, "Impulse"=w395:i32)
          n220 = Build Array(w401, w400, w399, w398, w397) -> (w396:dbl[])
        }
        n221 = Array Size(array=w363) -> (size(s)=w364:i32[])
        n222 = call-poly <userlib>:"Remove Duplicates from 1D Array__ogtk.vi"("Input Array"=w360) -> ("Output Array"=w361:i32[])  [unwired: 1 out]
        n223 = Index Array(array=w364) -> (element=w358:i32)  [unwired: 1 in]
        n224 = Array Size(array=w361) -> (size(s)=w359:i32)
        n225 = Equal To 0?(x=w358) -> (x = 0?=w362:bool)